vi "Joystick and Camera for pattern recognition.vi"(7 "controller in":T1={"A3200.lvclass"=refnum, "Ultimus V2.lvclass"=refnum, "NI-DAQ.lvclass"=refnum, "Motion.lvclass"=refnum, "I-O.lvclass"=refnum, "Dispenser.lvclass"=refnum}, 8 "XYZTheta":dbl[](array[numeric])=[0.026824843572167727, 0.5881986116746664, 0.00020513005945090647, -7.5327256914222e-06], 10 "I-O in":refnum<class "I-O.lvclass">, 11 "Motion in":refnum<class "Motion.lvclass">=refnum) -> (1 "Gantry":dbl[](array[numeric])=[737.9205478380792, 258.97431391859806, 4.360317709278066, -7.264279053542213e-06] format="%#_8g", 2 "I-O out":refnum<class "I-O.lvclass">, 3 "Motion out":refnum<class "Motion.lvclass">, 5 "controller out":T1)   [LabVIEW 2016]
uses:
  Classes/Controller/Camera/Camera Folder/Machine Vision.ctl
  Classes/Controller/Motion/Motion Folder/Motion.lvclass
  Classes/Controller/Motion/A3200 Folder/A3200.lvclass
  D:/Gantry_General/Classes/Controller/Motion/Motion Folder/Motion.lvclass
  Classes/Controller/I-O/I-O Folder/I-O.lvclass
  Classes/Controller/Dispenser/Ultimus V2 Folder/Ultimus V2.lvclass
  Classes/Controller/I-O/NI-DAQ Folder/NI-DAQ.lvclass
  D:/Gantry_General/Classes/Controller/I-O/I-O Folder/I-O.lvclass
  Classes/Controller/Dispenser/Dispenser Folder/Dispenser.lvclass
  <vilib>/Utility/file.llb/Write Delimited Spreadsheet (DBL).vi
  <vilib>/Utility/file.llb/Read Delimited Spreadsheet (DBL).vi
  Classes/Controller/Camera/Camera Folder/Camera.lvclass
panel:
  in  "path":path=path "D:/Gantry_General/Main/ms_kao/center and angle/DATA/001.TXT"
  in  "SAVE":bool
  in  "input":dbl
  in  "Camera light":bool
  in  "Go 3":bool
  in  "file path (dialog if empty) 3":path
  out "Bellow offset":dbl[](array[numeric])
  out "Camera 2":dbl[](array[numeric])=[0.0, 0.0, 52.864847366341415, 0.003106741190800654] format="%#_8g"
  out "Camera 1":dbl[](array[numeric])=[0.0, 0.0, 52.864847366341415, 0.003106741190800654] format="%#_8g"
  out "Bellow position":dbl[](array[numeric])=[0.0, 0.0, 52.864847366341415, 0.003106741190800654] format="%#_8g"
  in  "Record 2":bool
  in  "Record 1":bool
  in  "Pickup & Rotate":bool
  in  "Write to file":bool
  out "XYZTheta Out":dbl[](array[numeric])
  out "Waveform Graph":dbl[](graph)
  out "Array 2":dbl[](array[numeric])
  out "Array":dbl[](array[numeric])
  out "Numeric":dbl
  out "Image 2":T2(plugin-control)
  in  "Machine Vision 2":T3=enum."None"
  in  "interval":dbl
  in  "focus":bool
  in  "On/Off":bool=TRUE
  in  "Vacuum":bool
  out "Record Times":i32
  in  "Channel":i32=20
  in  "Filename":path=path "test.lvm"
  in  "Record":bool
  in  "Go 2":bool
  in  "Z Go":bool
  in  "Position":dbl
  in  "Machine Vision":T3=enum."None"
  in  "Go":bool
  in  "Joystick":bool
  out "Sum":dbl[](array[numeric])=[737.9205478380792, 258.97431391859806, 4.360317709278066, -7.264279053542213e-06] format="%#_8g"
  in  "Stop":bool
  out "Image":T2(plugin-control)
  out "Camera":dbl[](array[numeric]) format="%#_8g"
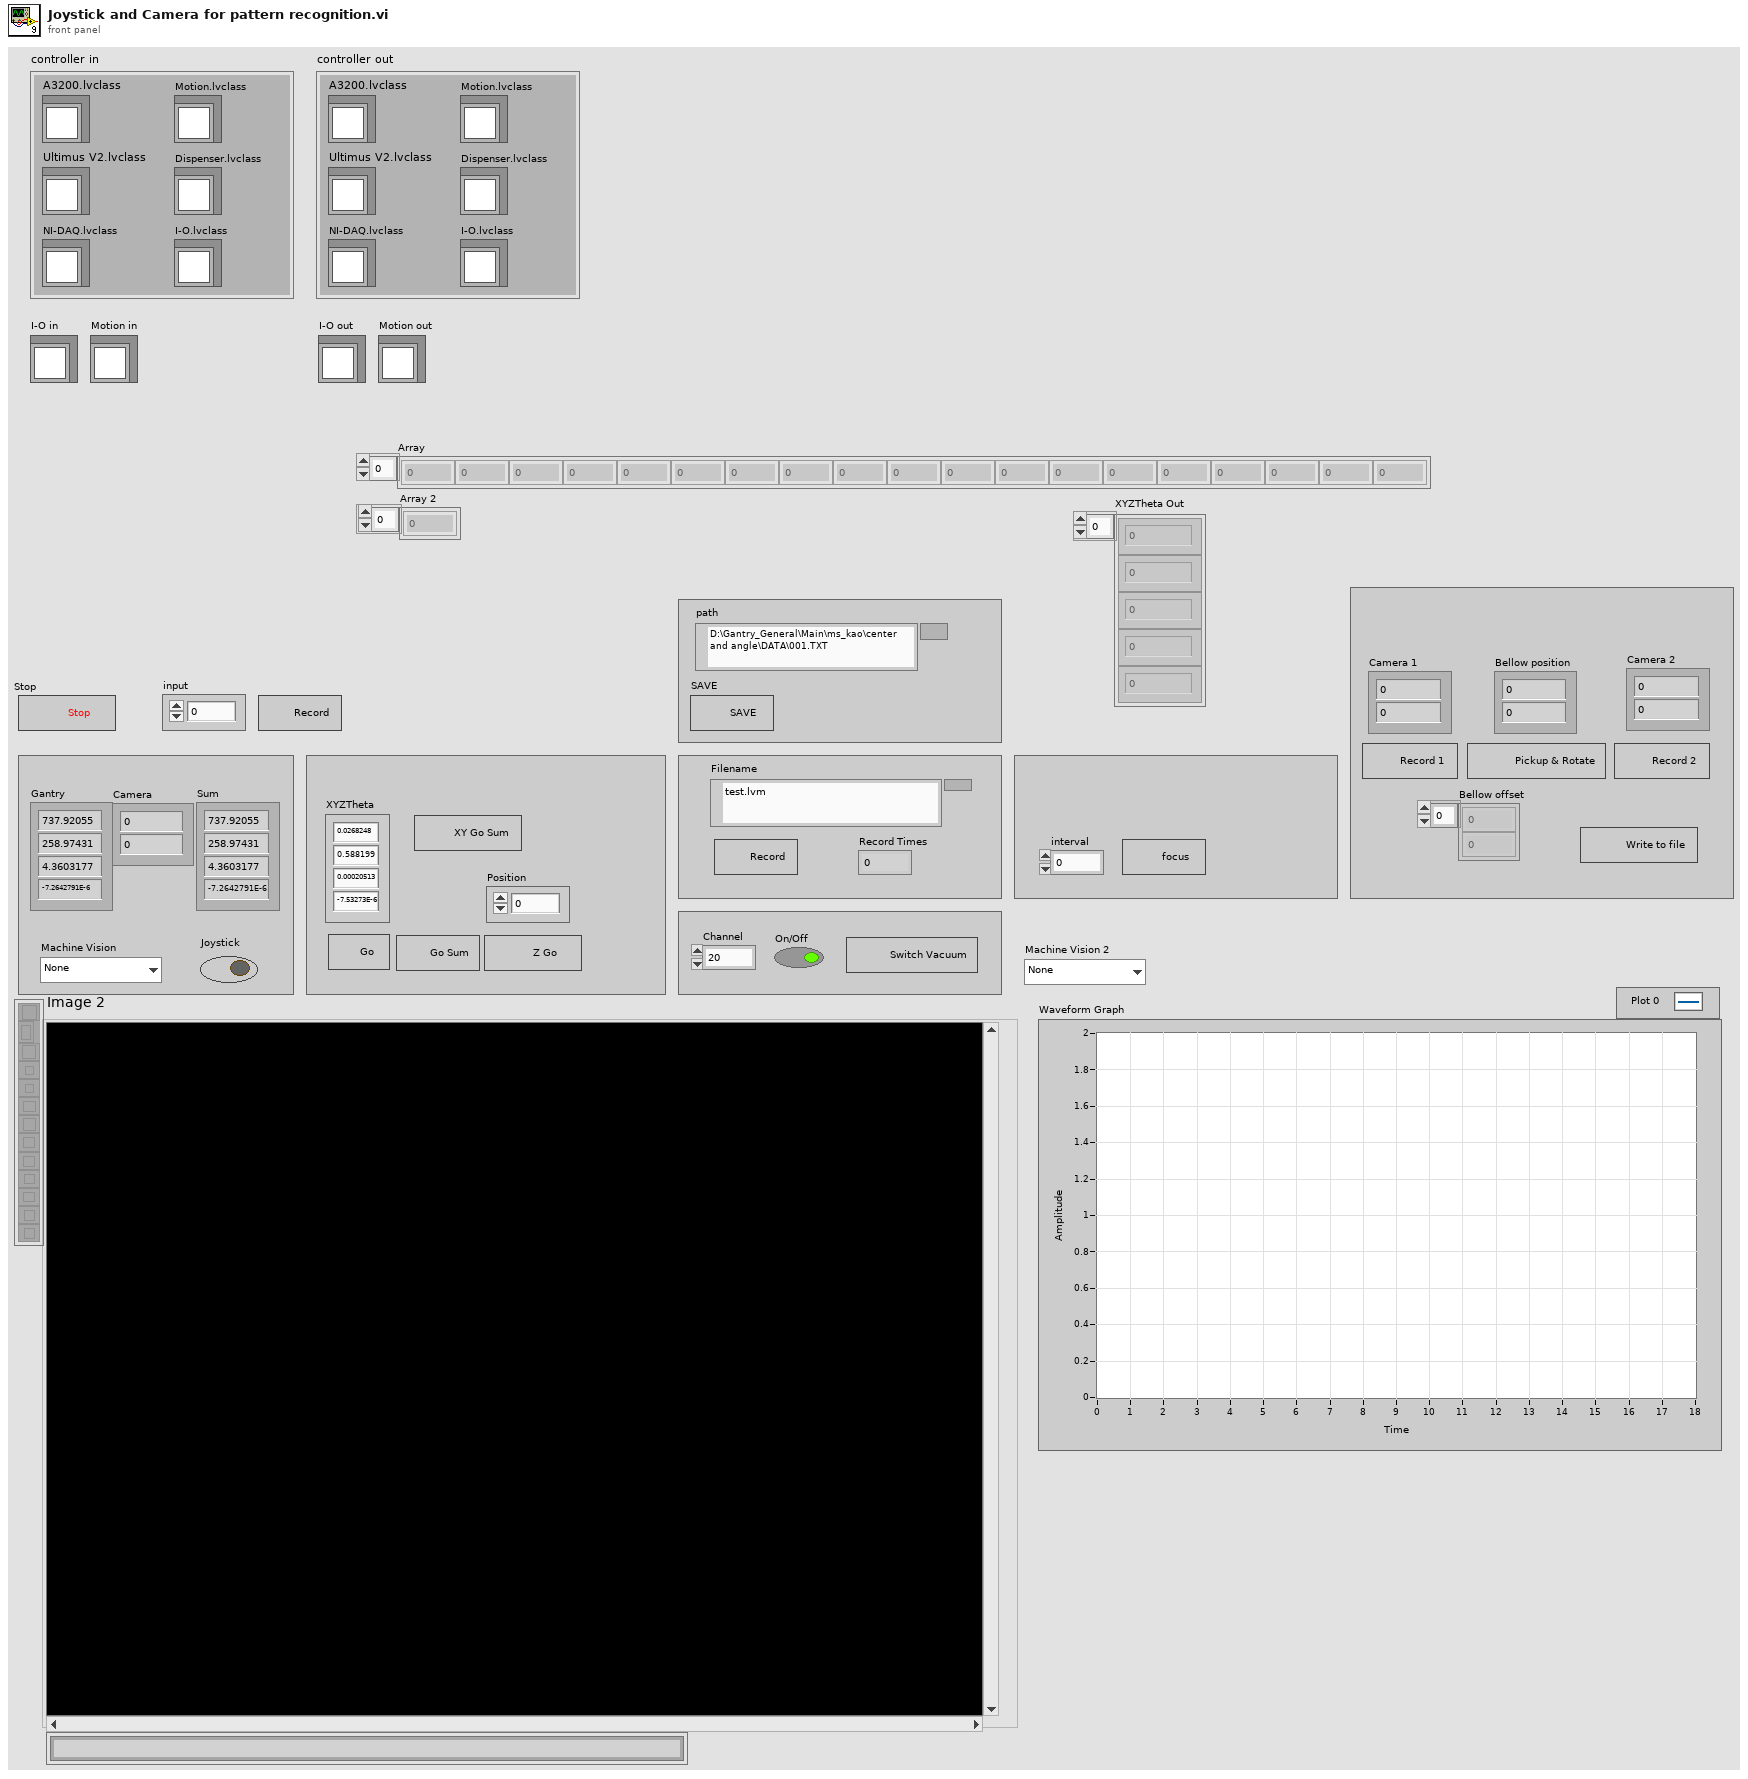
[diagram p1: front panel]
types:
  T1 = cluster{"A3200.lvclass":refnum<class "A3200.lvclass">, "Ultimus V2.lvclass":refnum<class "Ultimus V2.lvclass">, "NI-DAQ.lvclass":refnum<class "NI-DAQ.lvclass">, "Motion.lvclass":refnum<class "Motion.lvclass">, "I-O.lvclass":refnum<class "I-O.lvclass">, "Dispenser.lvclass":refnum<class "Dispenser.lvclass">}
  T2 = typedef "IMAQ Image.ctl" = refnum<image>
  T3 = typedef "Camera.lvclass/Machine Vision.ctl" = enum16{"top left corner", "top right corner", "bottom left corner", "bottom right corner", "bottom left chip", "top right chip", "None", "tracker fiducial", "chip cross 2", "chip cross", "Focus", "INTT HDI Mark", "INTT Sensor Cross", "INTT Chip Corner", "HPK Silicon", "HPK Silicon square", "8inch PCB Pad ", "8inch PCB Pad2", "Circle", "tpcb_hole"}
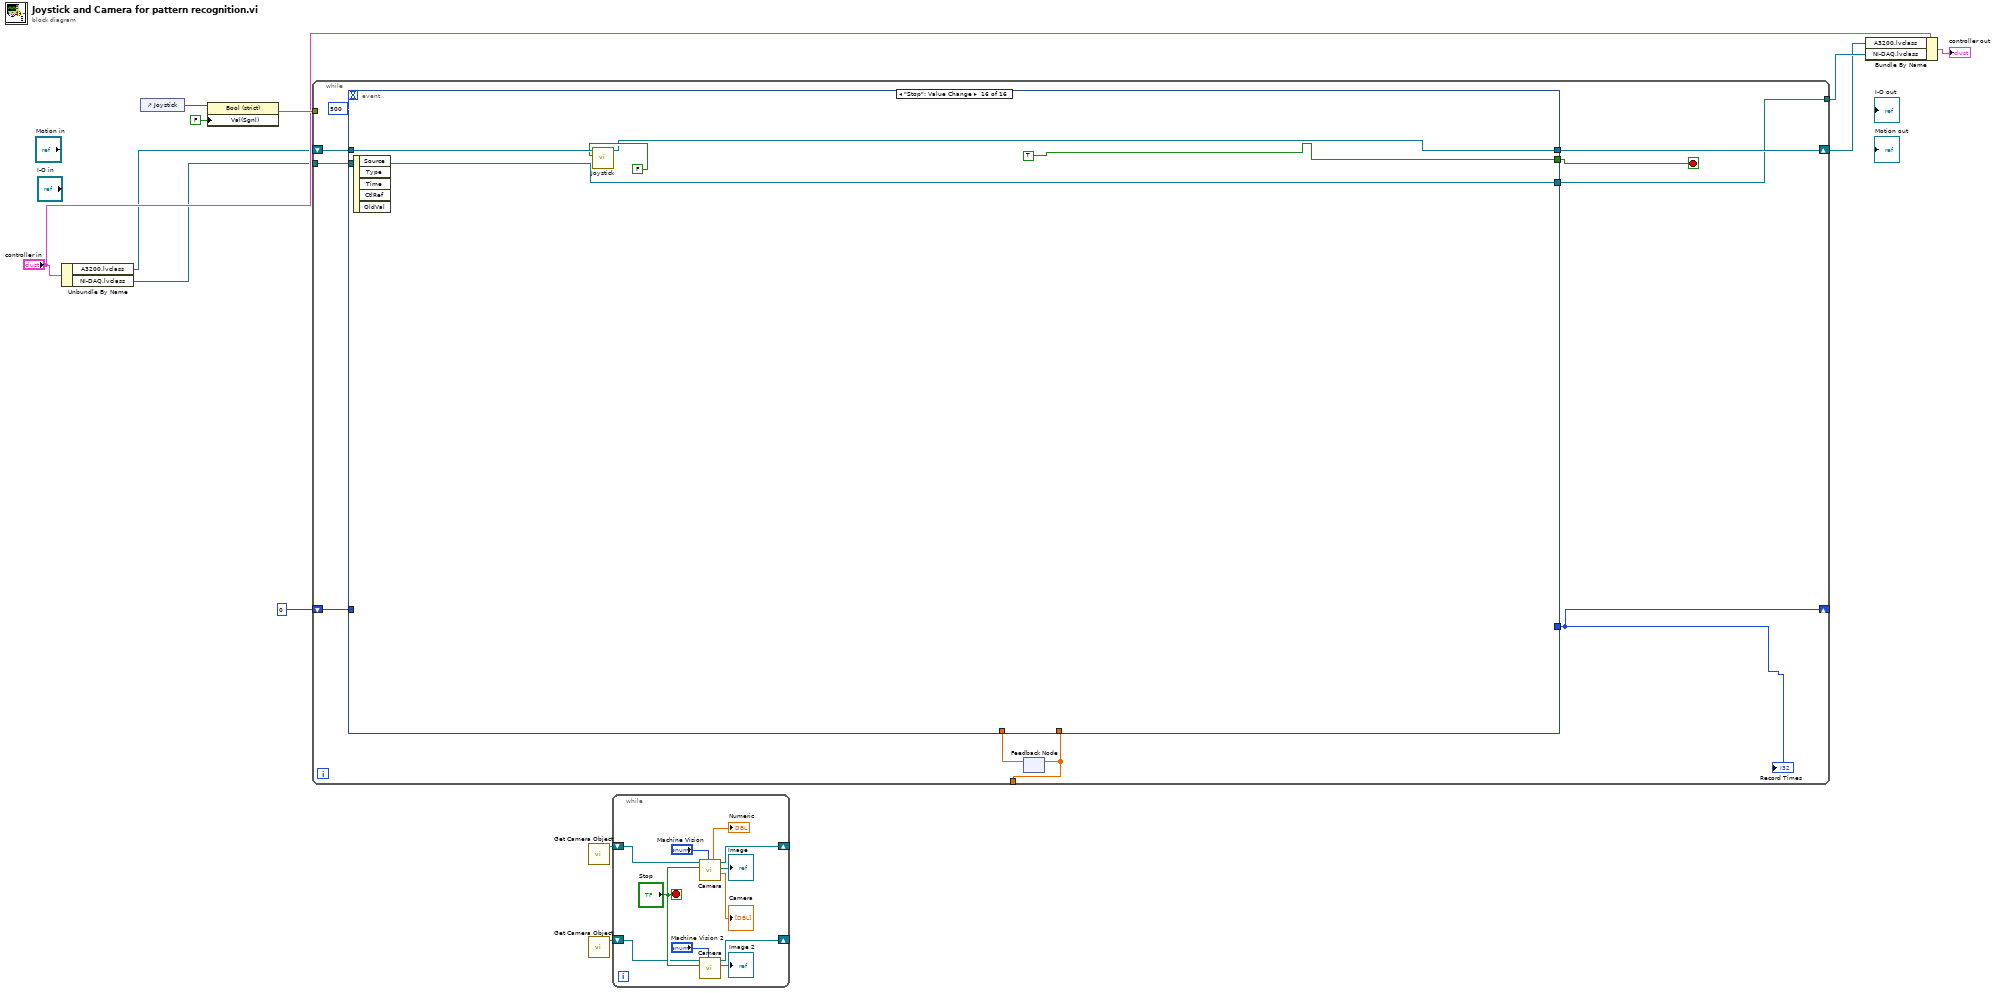
[diagram p0: block diagram]
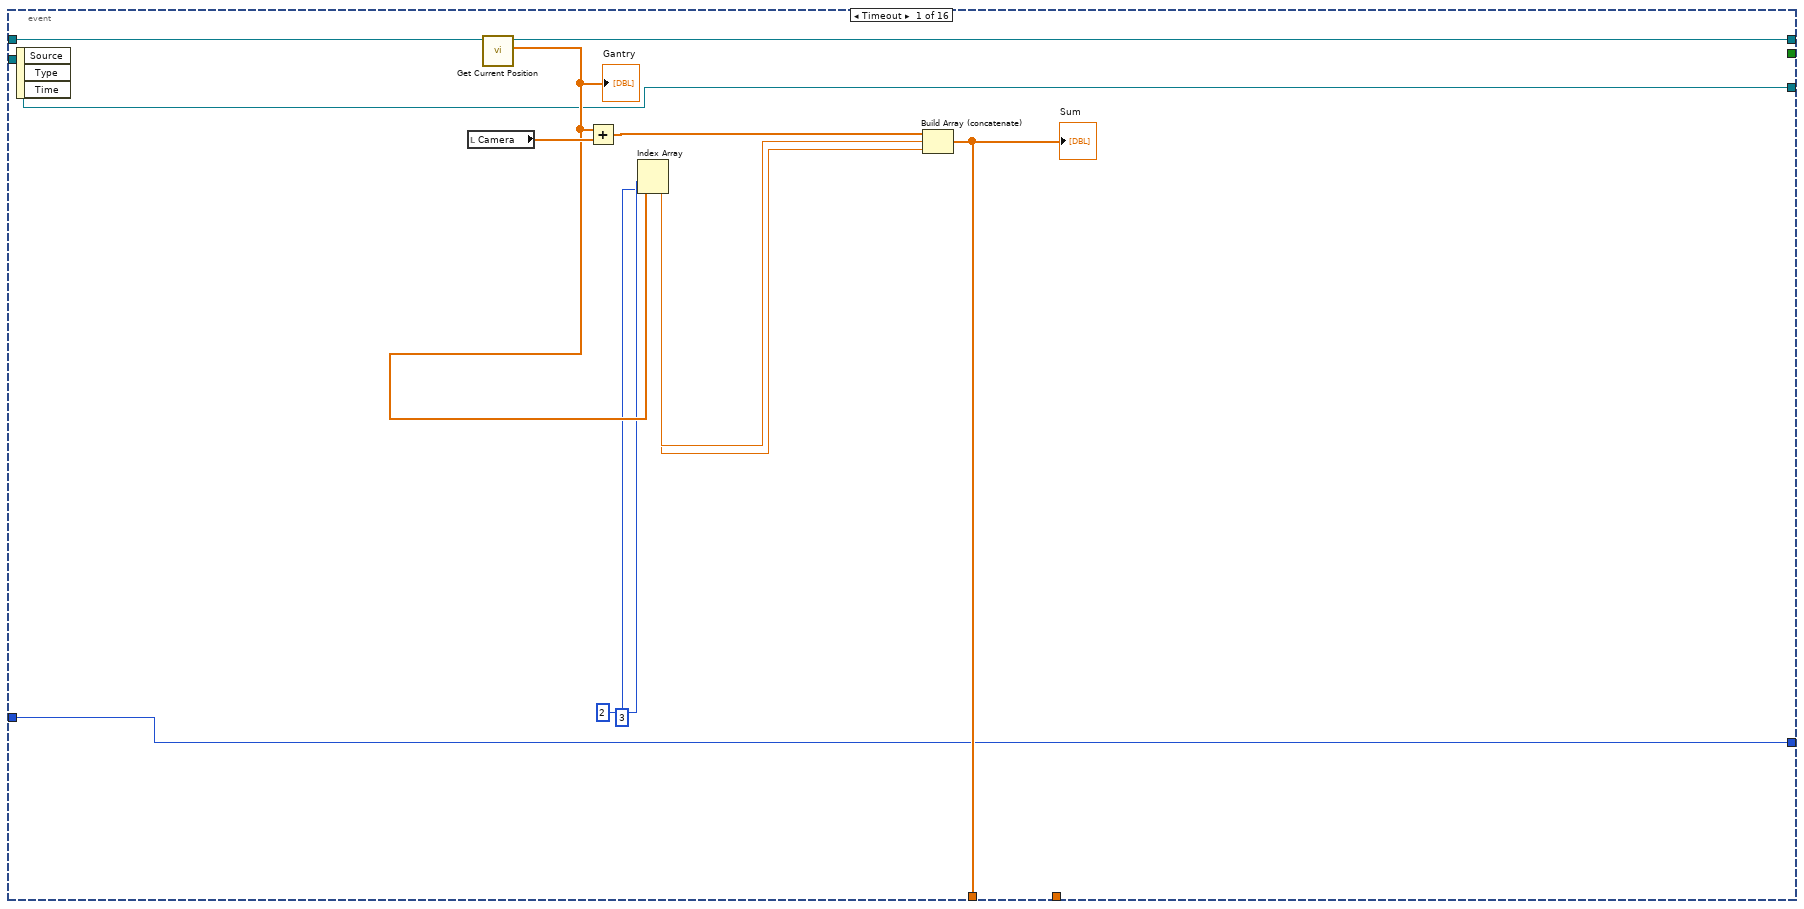
[diagram p2: hidden frame]
diagram:
  n1 = Unbundle By Name("controller in") -> ("A3200.lvclass"=w2:refnum<class "A3200.lvclass">, "NI-DAQ.lvclass"=w1:refnum<class "NI-DAQ.lvclass">)
  n2 = control-ref of="Joystick"() -> (w11:refnum<vi>)
  n3 = property class="Bool (strict)"(reference=w11, "Val(Sgnl)"=FALSE ("Value (Signaling)")) -> (error out=w10:errorcluster)  [unwired: 1 in, 1 out]
  n4 = while {
    shift-right: [w20] -> w3
    shift-left: w2 -> [w17]
    tunnel: w10 -> [_]
    tunnel: [w19] -> _
    tunnel: w1 -> [w14]
    shift-right: [w15] -> _
    shift-left: 0 -> [w16]
    tunnel: [w13] -> w4
    stop <- w21 stop-if-true
    n5 = feedback #1() -> (w19:dbl[])  [unwired: 1 in]
    n6 = event shown="[15] \"Stop\": Value Change" {
      selector: _ -> [_ _ _ _ _ _ _ _ _ _ _ _ _ _ _ _]
      dyn-events: _ -> [_ _ _ _ _ _ _ _ _ _ _ _ _ _ _ _]
      timeout: 500 -> [_ _ _ _ _ _ _ _ _ _ _ _ _ _ _ _]
      tunnel: [_ _ _ _ _ _ _ _ _ _ _ _ _ _ _ TRUE] -> w21
      tunnel: w17 -> [w33 w39 w44 w66 w80 w100 w111 w117 w127 w178 w184 w188 w201 w226 w242 w246]
      tunnel: [w32 w37 w43 w65 w79 w106 w111 w116 w135 w178 w184 w188 w201 w215 w242 w244] -> w20
      tunnel: [w28 _ _ _ _ _ _ _ _ _ _ _ _ _ _ _] -> w18
      tunnel: w19 -> [_ _ _ w63 w76 _ w113 _ _ _ _ _ _ _ _ _]
      tunnel: w16 -> [w24 w36 w41 w62 w77 w103 w109 _ _ _ _ _ _ _ w240 _]
      tunnel: [w24 w36 w41 w62 w77 w103 w108 _ _ _ _ _ _ _ w240 _] -> w15
      tunnel: w14 -> [w23 w35 w40 w61 w73 w102 w107 w123 w124 w182 w183 w187 w200 w224 w241 w243]
      tunnel: [w23 w35 w40 w61 w73 w102 w107 w123 w124 w181 w183 w187 w200 w208 w241 w243] -> w13
      event Timeout {
        n7 = event-data() -> ()  [unwired: 1 in, 3 out]
        n8 = local read "Camera"() -> (w34:dbl[])
        n9 = call-dynamic "Get Current Position.vi"("Gantry in"=w33) -> ("XYZTheta Out"=w30:dbl[], "Gantry out"=w32:refnum<class "A3200.lvclass">)  [unwired: 8 in, 1 out]
        "Gantry" <- w30
        n10 = Add(x=w30, y=w34) -> (x+y=w31:dbl[])
        n11 = Index Array(array=w30, index #1=2 ("index"), index #2=3 ("index")) -> (element #1=w26:dbl, element #2=w25:dbl)
        n12 = Build Array (concatenate)(w31, w26, w25) -> (w28:dbl[])
        "Sum" <- w28
      }
      event "Joystick": Value Change {
        n13 = event-data() -> ()  [unwired: 1 in, 6 out]
        n14 = call-dynamic "Joystick.vi"("Joystick"="Joystick", "Gantry in"=w39) -> ("Gantry out"=w37:refnum<class "A3200.lvclass">)  [unwired: 8 in, 1 out]
      }
      event "Go": Value Change {
        n15 = event-data() -> ()  [unwired: 1 in, 6 out]
        n16 = flat-sequence {
          tunnel: w44 -> [w46]
          tunnel: [w45] -> w42
          tunnel: [w48] -> w43
          tunnel: w42 -> [w51]
          frame #0 {
            n17 = call-dynamic "Joystick.vi"("Joystick"=FALSE, "Gantry in"=w46) -> ("Gantry out"=w45:refnum<class "A3200.lvclass">)  [unwired: 8 in, 1 out]
          }
          frame #1 {
            n18 = for {
              tunnel: "XYZTheta" -> [w58] mode=indexing
              tunnel: [w56] -> w50 mode=indexing
              shift-right: [w54] -> w49
              shift-left: w51 -> [w55]
              i -> [w60]
              n19 = Equal To 0?(x=w58) -> (x = 0?=w59:bool)
              n20 = call-dynamic "Get Current Position.vi"("Gantry in"=w55) -> ("XYZTheta Out"=w53:dbl[], "Gantry out"=w54:refnum<class "A3200.lvclass">)  [unwired: 8 in, 1 out]
              n21 = Index Array(array=w53, index=w60) -> (element=w57:dbl)
              n22 = Select(t=w57, s=w59, f=w58) -> (s? t:f=w56:dbl)
            }
            n23 = call "XYZTheta Go.vi"("XYZTheta In"=w50, "Motion in"=w49) -> ("Motion out"=w48:refnum<class "A3200.lvclass">)  [unwired: 7 in, 2 out]
          }
        }
      }
      event "Go 2": Value Change {
        n24 = event-data() -> ()  [unwired: 1 in, 6 out]
        n25 = flat-sequence {
          tunnel: w66 -> [w68]
          tunnel: [w67] -> w64
          tunnel: [w72] -> w65
          tunnel: w64 -> [w71]
          tunnel: w63 -> [w70]
          frame #0 {
            n26 = call-dynamic "Joystick.vi"("Joystick"=FALSE, "Gantry in"=w68) -> ("Gantry out"=w67:refnum<class "A3200.lvclass">)  [unwired: 8 in, 1 out]
          }
          frame #1 {
            n27 = call "XYZTheta Go.vi"("XYZTheta In"=w70, "Motion in"=w71) -> ("Motion out"=w72:refnum<class "A3200.lvclass">)  [unwired: 7 in, 2 out]
          }
        }
      }
      event "Go 3": Value Change {
        n28 = event-data() -> ()  [unwired: 1 in, 6 out]
        n29 = flat-sequence {
          tunnel: w80 -> [w82]
          tunnel: [w81] -> w78
          tunnel: [w92] -> w79
          tunnel: w78 -> [w93]
          tunnel: w74 -> [w84]
          frame #0 {
            n30 = call-dynamic "Joystick.vi"("Joystick"=FALSE, "Gantry in"=w82) -> ("Gantry out"=w81:refnum<class "A3200.lvclass">)  [unwired: 8 in, 1 out]
          }
          frame #1 {
            n31 = Index Array(array=w84) -> (element #1=w91:dbl, element #2=w89:dbl)  [unwired: 2 in]
            n32 = Greater?(x=w91, y=0.5) -> (0:w87:bool)
            n33 = Greater?(x=w89, y=0.5) -> (0:w86:bool)
            n34 = And(x=w87, y=w86) -> (x .and. y?=w85:bool)
            n35 = case shown="True" w85 {
              tunnel: w93 -> [w94 w98]
              tunnel: [w94 w97] -> w92
              tunnel: w84 -> [_ w95]
              frame False {
              }
              frame True {
                n36 = call-dynamic "Absolute XY Go.vi"("Speed"=20.0, "XY"=w95, "Gantry in"=w98) -> ("Gantry out"=w97:refnum<class "A3200.lvclass">)  [unwired: 7 in, 1 out]
              }
            }
          }
        }
        n37 = Delete From Array(array=w76, length=2) -> (array with subset deleted=w74:dbl[])  [unwired: 1 in, 1 out]
      }
      event "Z Go": Value Change {
        n38 = event-data() -> ()  [unwired: 1 in, 6 out]
        n39 = call-dynamic "Joystick.vi"("Joystick"=FALSE, "Gantry in"=w100) -> ("Gantry out"=w101:refnum<class "A3200.lvclass">)  [unwired: 8 in, 1 out]
        n40 = call-dynamic "Z Go.vi"("Speed"=2.0, "Position"="Position", "Gantry in"=w101) -> ("Gantry out"=w106:refnum<class "A3200.lvclass">)  [unwired: 7 in, 1 out]
      }
      event "Record": Value Change {
        n41 = event-data() -> ()  [unwired: 1 in, 6 out]
        n42 = Increment(x=w109) -> (x+1=w108:i32)
        n43 = call-poly <vilib>:"Write Delimited Spreadsheet.vi"("file path (dialog if empty)"="Filename", "format (%.3f)"="%.4f", "1D data"=w113, "append to file? (new file:F)"=TRUE) -> ()  [unwired: 10 in, 2 out]
      }
      event "SAVE": Value Change {
        n44 = event-data() -> ()  [unwired: 1 in, 6 out]
        n45 = call-dynamic "Get Current Position.vi"("Gantry in"=w117) -> ("XYZTheta Out"=w115:dbl[], "Gantry out"=w116:refnum<class "A3200.lvclass">)  [unwired: 8 in, 1 out]
        n46 = call "f_create file.vi"("path"="path") -> ("dup path"=w119:path)  [unwired: 10 in]
        n47 = call-poly <vilib>:"Read Delimited Spreadsheet.vi"("file path (dialog if empty)"=w119) -> ("new file path (Not A Path if cancelled)"=w120:path, "all rows"=w122:dbl[][])  [unwired: 9 in, 4 out]
        n48 = Build Array (concatenate)(w122, w115) -> (w121:dbl[][])
        n49 = call-poly <vilib>:"Write Delimited Spreadsheet.vi"("file path (dialog if empty)"=w120, "2D data"=w121) -> ()  [unwired: 12 in, 2 out]
      }
      event "focus": Value Change {
        (unwired) FALSE ("Joystick")
        n50 = event-data() -> ()  [unwired: 1 in, 6 out]
        n51 = call-dynamic "Joystick.vi"("Gantry in"=w127) -> ("Gantry out"=w126:refnum<class "A3200.lvclass">)  [unwired: 9 in, 1 out]
        n52 = Multiply(x="interval", y=-10) -> (x*y=w143:dbl)
        n53 = Build Array(w143) -> (w145:dbl[])
        n54 = call-dynamic "wrtCurrent Go.vi"("axis names"=string[] ["Z"] ("Axis"), "Speed"=10.0, "distances"=w145, "A3200 in"=w126) -> ("A3200 out"=w149:refnum<class "A3200.lvclass">)  [unwired: 6 in, 1 out]
        n55 = for {
          N: 19 -> [_]
          tunnel: w149 -> [w152]
          tunnel: [w156] -> w134
          shift-right: [w153] -> w141
          shift-left: dbl[] [] -> [w154]
          tunnel: "interval" -> [w159]
          tunnel: [w155] -> _
          n56 = for {
            N: 7 -> [_]
            shift-right: [w173] -> w164
            shift-left: dbl[] [] -> [w172]
            n57 = flat-sequence {
              tunnel: w172 -> [w175]
              tunnel: [w176] -> w171
              tunnel: [w177] -> w173
              tunnel: w171 -> [w177]
              frame #0 {
                n58 = local read "Numeric"() -> (w174:dbl)
                n59 = Insert Into Array(array=w175, new element=w174) -> (w176:dbl[])  [unwired: 1 in]
              }
              frame #1 {
                n60 = call "Time Delay2"() -> ()  [unwired: 11 in, 1 out]
              }
            }
          }
          n61 = call-dynamic "Get Current Position.vi"("Gantry in"=w152) -> ("XYZTheta Out"=→"XYZTheta Out":dbl[])  [unwired: 8 in, 2 out]
          n62 = Build Array(w159) -> (w158:dbl[])
          n63 = call-dynamic "wrtCurrent Go.vi"("axis names"=string[] ["Z"] ("Axis"), "Speed"=10.0, "distances"=w158, "A3200 in"=w152) -> ("error out"=w165:errorcluster, "A3200 out"=w156:refnum<class "A3200.lvclass">)  [unwired: 6 in]
          n64 = call "Convert to Dynamic Data"("Array"=w164) -> ("Dynamic Data Type"=w163:dynamicdata)  [unwired: 3 in]
          n65 = call "Statistics"("Signals"=w163) -> ("Arithmetic Mean"=w161:dynamicdata)  [unwired: 25 in, 1 out]
          n66 = call "Time Delay"("error in (no error)"=w165) -> ("error out"=w155:errorcluster)  [unwired: 10 in]
          n67 = call "Convert from Dynamic Data"("Dynamic Data Type"=w161) -> ("Array"=w157:dbl[])  [unwired: 3 in]
          n68 = for {
            tunnel: w157 -> [w170] mode=indexing
            shift-right: [w169] -> w153
            shift-left: w154 -> [w168]
            n69 = Insert Into Array(array=w168, new element=w170) -> (w169:dbl[])  [unwired: 1 in]
          }
          "Array" <- w153
          "Waveform Graph" <- w153
        }
        n70 = call "Convert to Dynamic Data2"("Array"=w141) -> ("Dynamic Data Type"=w140:dynamicdata)  [unwired: 3 in]
        n71 = call "Statistics2"("Signals"=w140) -> ("Index of Max"=w139:dynamicdata)  [unwired: 25 in, 1 out]
        n72 = call "Convert from Dynamic Data2"("Dynamic Data Type"=w139) -> ("Array"=w125:dbl[])  [unwired: 3 in]
        "Array 2" <- w125
        n73 = Index Array(array=w125, index=0) -> (element=w129:dbl)
        n74 = local read "interval"() -> (w132:dbl)
        n75 = Subtract(x=w129, y=18.0 ("x")) -> (x-y=w133:dbl)
        n76 = Multiply(x=w132, y=w133) -> (x*y=w131:dbl)
        n77 = Build Array(w131) -> (w130:dbl[])
        n78 = call-dynamic "wrtCurrent Go.vi"("axis names"=string[] ["Z"] ("Axis"), "Speed"=10.0, "distances"=w130, "A3200 in"=w134) -> ("A3200 out"=w135:refnum<class "A3200.lvclass">)  [unwired: 6 in, 1 out]
      }
      event "Vacuum": Value Change {
        n79 = event-data() -> ()  [unwired: 1 in, 6 out]
        n80 = call-dynamic "Digital Write 1 Channel.vi"("Value"="On/Off", "Channel"="Channel", "NI-DAQ.lvclass"=w182) -> ("NI-DAQ.lvclass 2"=w181:refnum<class "NI-DAQ.lvclass">)  [unwired: 7 in, 1 out]
      }
      event "Record 1": Value Change {
        n81 = event-data() -> ()  [unwired: 1 in, 6 out]
        n82 = local read "Gantry"() -> (→"Bellow position":dbl[])
        n83 = local read "Sum"() -> (→"Camera 1":dbl[])
      }
      event "Record 2": Value Change {
        n84 = event-data() -> ()  [unwired: 1 in, 6 out]
        n85 = local read "Sum"() -> (→"Camera 2":dbl[])
      }
      event "Write to file": Value Change {
        n86 = event-data() -> ()  [unwired: 1 in, 6 out]
        n87 = local read "Camera 1"() -> (w204:dbl[])
        n88 = local read "Camera 2"() -> (w203:dbl[])
        n89 = local read "Bellow position"() -> (w198:dbl[])
        n90 = Add(x=w204, y=w203) -> (x+y=w202:dbl[])
        n91 = Divide(x=w202, y=2.0) -> (x/y=w199:dbl[])
        n92 = Subtract(x=w198, y=w199) -> (x-y=w197:dbl[])
        n93 = Index Array(array=w197, index #1=0 ("index"), index #2=1 ("index")) -> (element #1=w194:dbl, element #2=w193:dbl)
        n94 = Build Array(w194, w193, 0.0 ("element"), 0.0 ("element")) -> (w190:dbl[])
        "Bellow offset" <- w190
        n95 = call-poly <vilib>:"Write Delimited Spreadsheet.vi"("file path (dialog if empty)"="file path (dialog if empty) 3", "1D data"=w190, "append to file? (new file:F)"=FALSE) -> ()  [unwired: 11 in, 2 out]
      }
      event "Pickup & Rotate": Value Change {
        n96 = event-data() -> ()  [unwired: 1 in, 6 out]
        n97 = call-dynamic "Joystick.vi"("Joystick"=FALSE, "Gantry in"=w226) -> ("Gantry out"=w225:refnum<class "A3200.lvclass">)  [unwired: 8 in, 1 out]
        n98 = call "Lower_Stop.vi"("I-O in"=w224, "Motion in"=w225) -> ("I-O out"=w223:refnum<class "NI-DAQ.lvclass">, "Motion out"=w222:refnum<class "A3200.lvclass">)  [unwired: 7 in, 1 out]
        n99 = call "WriteReadWait.vi"("Read Value"=TRUE, "Write Value"=TRUE, "Read"=1, "Write"=1, "I-O in"=w223) -> ("error out"=w233:errorcluster, "I-O out"=w221:refnum<class "NI-DAQ.lvclass">)  [unwired: 5 in]
        n100 = call-dynamic "wrtCurrent Go.vi"("axis names"=string[] ["Z"] ("Axis"), "error in (no error)"=w233, "Speed"=10.0, "distances"=dbl[] [-20.0] ("Distance"), "A3200 in"=w222) -> ("A3200 out"=w230:refnum<class "A3200.lvclass">)  [unwired: 5 in, 1 out]
        n101 = call-dynamic "wrtCurrent Go.vi"("axis names"=string[] ["U"] ("Axis"), "Speed"=10.0, "distances"=dbl[] [180.0] ("Distance"), "A3200 in"=w230) -> ("A3200 out"=w220:refnum<class "A3200.lvclass">)  [unwired: 6 in, 1 out]
        n102 = call "Lower_Stop.vi"("I-O in"=w221, "Motion in"=w220) -> ("I-O out"=w209:refnum<class "NI-DAQ.lvclass">, "Motion out"=w216:refnum<class "A3200.lvclass">)  [unwired: 7 in, 1 out]
        n103 = call-dynamic "wrtCurrent Go.vi"("axis names"=string[] ["Z"] ("Axis"), "Speed"=10.0, "distances"=dbl[] [-20.0] ("Distance"), "A3200 in"=w216) -> ("A3200 out"=w215:refnum<class "A3200.lvclass">)  [unwired: 6 in, 1 out]
        n104 = call "WriteReadWait.vi"("Read Value"=FALSE, "Write Value"=FALSE, "Read"=1, "Write"=1, "I-O in"=w209) -> ("I-O out"=w208:refnum<class "NI-DAQ.lvclass">)  [unwired: 5 in, 1 out]
      }
      event "Camera light": Value Change {
        n105 = event-data() -> ()  [unwired: 1 in, 6 out]
        n106 = call "Camera Light.vi"("input"="input") -> ()  [unwired: 2 in, 1 out]
      }
      event "Stop": Value Change {
        n107 = event-data() -> ()  [unwired: 1 in, 5 out]
        n108 = call-dynamic "Joystick.vi"("Joystick"=FALSE, "Gantry in"=w246) -> ("Gantry out"=w244:refnum<class "A3200.lvclass">)  [unwired: 8 in, 1 out]
      }
    }
    "Record Times" <- w15
    n109 = feedback-in #1(w18) -> ()
  }
  n110 = call "Get Camera Object.vi"() -> ("Camera out"=w9:refnum<class "Camera.lvclass">)  [unwired: 10 in, 1 out]
  n111 = call "Get Camera Object.vi"() -> ("Camera out"=w7:refnum<class "Camera.lvclass">)  [unwired: 10 in, 1 out]
  n112 = while {
    shift-right: [w257] -> _
    shift-left: w9 -> [w258]
    shift-right: [w250] -> _
    shift-left: w7 -> [w251]
    stop <- "Stop" stop-if-true
    n113 = call "Camera.vi"("Machine Vision"="Machine Vision", "Stop"="Stop", "Camera in"=w258) -> ("Camera"=→"Camera":dbl[], "Image"=→"Image":T2, "Camera out"=w257:refnum<class "Camera.lvclass">, "Focus output"=→"Numeric":dbl)  [unwired: 4 in, 1 out]
    n114 = call "Camera.vi"("Machine Vision"="Machine Vision 2", "Stop"="Stop", "Camera in"=w251) -> ("Image"=→"Image 2":T2, "Camera out"=w250:refnum<class "Camera.lvclass">)  [unwired: 4 in, 3 out]
  }
  n115 = Bundle By Name(cluster="controller in", "A3200.lvclass"=w3, "NI-DAQ.lvclass"=w4) -> (→"controller out":T1)